vi "UHR-Fleezers Control (host) - 12.7c.vi"() -> ()   [LabVIEW 2012] (continued)
                n1635 = local write "Set Confocal Spot (X-Y)"(w2359) -> ()
                n1636 = local write "Set X Only"(w2359) -> ()
                n1637 = local write "Set Y Only"(w2359) -> ()
              }
            }
          }
          frame 3 {
            n1638 = local read "BD 2 Frequency 1 (MHz)"() -> (w2395:dbl)
            n1639 = local read "BD 1 Frequency 1 (MHz)"() -> (w2396:dbl)
            n1640 = local write "Manipulating Trap"(TRUE ("Manipulating Trap")) -> ()
            n1641 = local write "Coords"(T7 {"Horizontal"=0, "Vertical"=0} ("Coords")) -> ()
            n1642 = while {
              tunnel: w2401 -> [w2406]
              tunnel: w2399 -> [w2405]
              tunnel: w2397 -> [w2404]
              tunnel: w2396 -> [w2403]
              tunnel: w2395 -> [w2402]
              stop <- w2407 stop-if-true
              n1643 = event shown="[0] \"Pane\": Mouse Move" {
                selector: _ -> [_ _]
                dyn-events: _ -> [_ _]
                timeout: _ -> [_ _]
                tunnel: ["Force Manip Abort" w2471] -> w2407
                tunnel: w2406 -> [w2414 _]
                tunnel: w2405 -> [w2412 _]
                tunnel: w2404 -> [w2411 _]
                tunnel: w2403 -> [w2410 _]
                tunnel: w2402 -> [w2409 _]
                event Mouse Move {
                  n1644 = event-data() -> ("Time"=w2415:u32, "Coords"=w2416:T7)  [unwired: 3 out]
                  n1645 = Less?(x=w2415, y=w2414) -> (x < y?=w2413:bool)
                  n1646 = case "Makes sure old motion events prior to mouse click aren't used" shown="False" w2413 {
                    tunnel: w2416 -> [w2458 _]
                    tunnel: w2412 -> [w2459 _]
                    tunnel: w2411 -> [w2436 _]
                    tunnel: w2410 -> [w2432 _]
                    tunnel: w2409 -> [w2431 _]
                    frame False {
                      n1647 = Subtract(x=w2458, y=w2459) -> (x-y=w2457:T7)
                      "Coords" <- w2457
                      n1648 = local read "Y RF Frequency Limits (MHz)"() -> (w2417:T16)
                      n1649 = To Double Precision Float(number=w2457) -> (double precision float=w2456:cluster{"Horizontal":dbl, "Vertical":dbl})
                      n1650 = Multiply(x=cluster{"Horizontal":dbl, "Vertical":dbl} {"Horizontal"=-1.0, "Vertical"=1.0}, y="Manipulation Scaling") -> (x*y=w2452:cluster{"Horizontal":dbl, "Vertical":dbl})
                      n1651 = local read "X RF Frequency Limits (MHz)"() -> (w2418:T16)
                      n1652 = Multiply(x=w2456, y=w2452) -> (x*y=w2454:cluster{"Horizontal":dbl, "Vertical":dbl})
                      n1653 = Unbundle By Name(w2454) -> ("Horizontal"=w2449:dbl, "Vertical"=w2453:dbl)
                      n1654 = Unbundle By Name(w2417) -> ("Maximum"=w2420:dbl, "Minimum"=w2419:dbl)
                      n1655 = Boolean To (0,1)(Boolean="Manip. X?") -> (0, 1=w2447:i16)
                      n1656 = Boolean To (0,1)(Boolean="Manip. Y?") -> (0, 1=w2444:i16)
                      n1657 = local read "BD 1 Frequency 2 (MHz)"() -> (w2434:dbl)
                      n1658 = Multiply(x=w2453, y=w2444) -> (x*y=w2446:dbl)
                      n1659 = Multiply(x=w2447, y=w2449) -> (x*y=w2450:dbl)
                      n1660 = local read "BD 2 Frequency 2 (MHz)"() -> (w2433:dbl)
                      n1661 = Unbundle By Name(w2418) -> ("Maximum"=w2422:dbl, "Minimum"=w2421:dbl)
                      n1662 = Add(x=w2431, y=w2446) -> (x+y=w2424:dbl)
                      n1663 = Add(x=w2432, y=w2450) -> (x+y=w2426:dbl)
                      n1664 = In Range and Coerce(upper limit=w2422, x=w2426, lower limit=w2421) -> (coerced(x)=w2425:dbl)  [unwired: 1 out]
                      n1665 = In Range and Coerce(upper limit=w2420, x=w2424, lower limit=w2419) -> (coerced(x)=w2423:dbl)  [unwired: 1 out]
                      n1666 = Subtract(x=w2425, y=w2434) -> (x-y=w2443:dbl)
                      n1667 = Subtract(x=w2423, y=w2433) -> (x-y=w2442:dbl)
                      n1668 = Square(x=w2443) -> (x^2=w2441:dbl)
                      n1669 = Square(x=w2442) -> (x^2=w2440:dbl)
                      n1670 = Add(x=w2441, y=w2440) -> (x+y=w2439:dbl)
                      n1671 = Square Root(x=w2439) -> (sqrt(x)=w2435:dbl)
                      n1672 = In Range and Coerce(upper limit="Limit Max (MHz)", x=w2435, lower limit="Limit Min (MHz)") -> (In Range?=w2428:bool)  [unwired: 1 out]
                      n1673 = Not(x="Limits Enable") -> (.not. x?=w2427:bool)
                      n1674 = Or(x=w2428, y=w2427) -> (x .or. y?=w2429:bool)
                      n1675 = case shown="True" w2429 {
                        tunnel: w2436 -> [_ w2469]
                        tunnel: w2435 -> [_ w2460]
                        tunnel: w2425 -> [_ w2467]
                        tunnel: w2434 -> [_ w2466]
                        tunnel: w2423 -> [_ w2465]
                        tunnel: w2433 -> [_ w2464]
                        tunnel: w2418 -> [_ w2462]
                        tunnel: w2417 -> [_ w2461]
                        frame False {
                        }
                        frame True {
                          n1676 = local read "BD 1 Frequency 3 (MHz)"() -> (w2468:dbl)
                          n1677 = local read "BD 2 Frequency 3 (MHz)"() -> (w2463:dbl)
                          n1678 = local write "Trap Delta (MHz)"(w2460) -> ()
                          n1679 = call "set RF board frequency - interlace.vi"("Board 2 Frequency Limits"=w2461, "Board 1 Frequency Limits"=w2462, "FPGA VI Reference In"=w2469, "Board 2 Frequency 3 (MHz)"=w2463, "Board 1 Frequency 3 (MHz)"=w2468, "Board 2 Frequency 2 (MHz)"=w2464, "Board 2 Frequency 1 (MHz)"=w2465, "Board 1 Frequency 2 (MHz)"=w2466, "Board 1 Frequency 1  (MHz)"=w2467) -> ()  [unwired: 1 in, 2 out]
                          n1680 = local write "BD 2 Frequency 1 (MHz)"(w2465) -> ()
                          n1681 = local write "BD 1 Frequency 1 (MHz)"(w2467) -> ()
                        }
                      }
                    }
                    frame True {
                    }
                  }
                }
                event Mouse Up {
                  n1682 = event-data() -> ("Button"=w2470:u16)  [unwired: 8 out]
                  n1683 = case shown="3" w2470 {
                    tunnel: [FALSE TRUE] -> w2471
                    frame 0, Default {
                    }
                    frame 3 {
                      n1684 = local read "Trap Delta (MHz)"() -> (w2473:dbl)
                      n1685 = property on="Initial delta (MHz)" class="DigNum (strict)"("Val(Sgnl)"=w2473) -> ()  [unwired: 2 in, 2 out]
                      n1686 = local write "Manipulating Trap"(FALSE ("Manipulating Trap")) -> ()
                    }
                  }
                }
              }
            }
          }
        }
      }
      event Mouse Move {
        n1687 = event-data() -> ()  [unwired: 6 out]
      }
    }
    n1688 = local read "Stop All"() -> (w2289:bool)
    n1689 = node-c288() -> ()  [unwired: 2 out]
  }
  n1690 = timed-loop "Run Scripts, including: stage motion" {
    tunnel: w125 -> [w2484]
    tunnel: w124 -> [w2485]
    tunnel: [w2485] -> w123
    tunnel: [w2484] -> w122
    timing: w120 -> [_]
    timing-out: [_] -> w119
    tunnel: w106 -> [w2483]
    tunnel: w107 -> [w2482]
    tunnel: w78 -> [w2479]
    tunnel: w77 -> [w2478]
    tunnel: w76 -> [w2480]
    tunnel: w75 -> [w2481]
    tunnel: w13 -> [w2477]
    tunnel: w1 -> [w2476]
    stop <- w2486 stop-if-true
    n1691 = node-c288() -> ()  [unwired: 1 in, 1 out]
    n1692 = event shown="[22] \"Move in a Circle\": Value Change" {
      selector: _ -> [_ _ _ _ _ _ _ _ _ _ _ _ _ _ _ _ _ _ _ _ _ _ _ _]
      dyn-events: _ -> [_ _ _ _ _ _ _ _ _ _ _ _ _ _ _ _ _ _ _ _ _ _ _ _]
      timeout: _ -> [_ _ _ _ _ _ _ _ _ _ _ _ _ _ _ _ _ _ _ _ _ _ _ _]
      tunnel: ["Set Position" "Move to Position" _ _ _ _ _ _ "Read Harvard" _ _ _ _ _ _ "Got ADig bead" "Force FB Data\nScript" _ "Got DNA bead" "Take Stepping Data" _ "Take Detection Laser\nImage" _ _] -> _
      tunnel: [_ _ _ _ _ _ _ _ _ _ _ _ _ _ _ _ _ _ _ _ _ _ _ w3274] -> w2486
      tunnel: w2484 -> [w2504 w2512 w2525 w2555 _ _ _ _ _ w2671 w2711 w2792 w2821 w2953 w2979 _ w3015 _ _ _ _ _ _ _]
      tunnel: w2485 -> [w2505 w2513 w2526 w2556 _ _ _ _ _ w2672 w2712 w2793 w2822 w2954 w2980 _ w3016 _ _ _ _ _ _ _]
      tunnel: w2483 -> [_ _ _ _ _ _ _ _ w2656 _ _ _ _ _ _ _ _ _ _ _ _ _ _ _]
      tunnel: w2482 -> [_ _ _ _ _ _ _ _ w2655 _ _ _ _ _ _ _ _ _ _ _ _ _ _ _]
      tunnel: w2481 -> [_ _ _ _ _ _ _ _ _ _ _ _ _ _ _ _ _ _ _ _ _ _ _ _]
      tunnel: w2480 -> [_ _ _ _ _ _ _ _ _ _ _ _ _ _ _ _ _ _ _ _ _ _ _ _]
      tunnel: w2479 -> [_ _ _ _ _ _ _ _ _ _ _ _ _ _ _ _ _ _ _ _ _ _ _ _]
      tunnel: w2478 -> [_ _ _ _ _ _ _ _ _ _ _ _ _ _ _ _ _ _ _ _ _ _ _ _]
      tunnel: w2477 -> [_ _ _ _ w2583 w2611 w2635 w2646 _ _ _ _ _ _ _ _ _ _ _ _ _ _ _ w3273]
      tunnel: w2476 -> [_ _ _ _ _ _ _ _ _ _ _ _ _ _ _ _ _ _ _ _ _ _ w3174 _]
      event "Set Position", "Set Position 2", "Set Position 3", "Set Position 4", "Set Position 5", "Set Position 1": Value Change {
        n1693 = event-data() -> ()  [unwired: 1 in, 5 out]
        n1694 = Build Array("Set Position 1", "Set Position 2", "Set Position 3", "Set Position 4", "Set Position 5") -> (w2503:bool[])
        n1695 = Boolean Array To Number(Boolean array=w2503) -> (number=w2502:u32)
        n1696 = Logarithm Base 2(1:w2502) -> (0:w2494:dbl)
        n1697 = call "Read Stage Position.vi"("error in"=w2504, "VISA resource name in"=w2505) -> ("Current Position"=w2509:cluster{dbl, dbl, dbl}, "error out"=w2508:errorcluster)  [unwired: 2 out]
        n1698 = Decrement(x="Position") -> (x-1=w2492:dbl)
        n1699 = Greater Or Equal?(x=w2494, y=0.0) -> (x >= y?=w2495:bool)
        n1700 = Cluster To Array(cluster=w2509) -> (array=w2506:dbl[])
        n1701 = local write "Stage Control Serial Error"(w2508) -> ()
        n1702 = Select(t=w2494, s=w2495, f=w2492) -> (s? t:f=w2491:dbl)
        n1703 = Increment(x=w2491) -> (x+1=w2490:dbl)
        n1704 = Build Array (concatenate)(w2490, w2506) -> (w2489:dbl[])
        n1705 = Replace Array Subset(array="Saved Stage Positions", new element=w2489, index (row)=w2491) -> (w2507:dbl[][])  [unwired: 1 in]
        n1706 = local write "Saved Stage Positions"(w2507) -> ()
      }
      event "Move to Position": Value Change {
        n1707 = event-data() -> ()  [unwired: 1 in, 5 out]
        n1708 = flat-sequence {
          tunnel: w2513 -> [w2517]
          tunnel: w2512 -> [w2516]
          frame #0 {
            n1709 = local read "Saved Stage Positions"() -> (w2519:dbl[][])
            n1710 = local read "Position"() -> (w2518:dbl)
            n1711 = local write "Stage Moving"(TRUE ("Stage Moving")) -> ()
            n1712 = call "move to saved stage position.vi"("error in"=w2516, "Stage VISA resource name in"=w2517, "Position"=w2518, "Saved Stage Positions"=w2519) -> ("error out"=w2515:errorcluster)  [unwired: 1 out]
            n1713 = local write "Stage Control Serial Error"(w2515) -> ()
          }
          frame #1 {
            n1714 = call <vilib>:"Beep.vi"() -> ()  [unwired: 3 in, 9 out]
            n1715 = local write "Stage Moving"(FALSE ("Stage Moving")) -> ()
          }
        }
      }
      event "Move Cap. 1 (DNA Bottom)": Value Change {
        n1716 = event-data() -> ()  [unwired: 1 in, 5 out]
        n1717 = local write "Move Cap. 1 (DNA Bottom)"(FALSE ("Move Cap. 1 (DNA Right)")) -> ()
        n1718 = flat-sequence {
          tunnel: w2525 -> [w2528]
          tunnel: w2526 -> [w2529]
          tunnel: [w2529] -> w2523
          tunnel: [w2528] -> w2522
          tunnel: w2523 -> [w2531]
          tunnel: w2522 -> [w2530]
          frame #0 {
            n1719 = property on="Sample Channel\nFlow" class="Bool (strict)"("Val(Sgnl)"="Cap 1 Samp Flow ON") -> ()  [unwired: 2 in, 2 out]
          }
          frame #1 {
            n1720 = local read "Saved Stage Positions"() -> (w2541:dbl[][])
            n1721 = local write "Stage Moving"(TRUE ("Stage Moving")) -> ()
            n1722 = Array Subset(array=w2541, index (row)=0 ("index"), length (row)=1 ("length"), index (col)=1 ("index"), length (col)=3 ("length")) -> (w2538:dbl[][])
            n1723 = Reshape Array(w2538, 3 ("dimension size")) -> (w2536:dbl[])
            n1724 = Array To Cluster(array=w2536) -> (cluster=w2535:cluster{"[0]":dbl, "[1]":dbl, "[2]":dbl})
            n1725 = call "Set Stage Position.vi"("Position"=w2535, "error in"=w2530, "VISA resource name in"=w2531) -> ("error out"=w2534:errorcluster)  [unwired: 2 out]
            n1726 = local write "Stage Control Serial Error"(w2534) -> ()
          }
          frame #2 {
            n1727 = local write "Stage Moving"(FALSE ("Stage Moving")) -> ()
            n1728 = case shown="True" "Cap 1 Flow ON" {
              frame False {
              }
              frame True {
                n1729 = property on="Inject Pump 1" class="Bool (strict)"("Val(Sgnl)"=TRUE ("Value (Signaling)")) -> ()  [unwired: 2 in, 2 out]
              }
            }
            n1730 = call <vilib>:"Beep.vi"() -> ()  [unwired: 3 in, 9 out]
          }
          frame #3 {
            n1731 = property on="Sample Channel\nFlow" class="Bool (strict)"("Val(Sgnl)"=FALSE ("Value (Signaling)")) -> ()  [unwired: 2 in, 2 out]
            n1732 = local read "Cap. 2 BD T1?\n(ADig T1, DNA T2)"() -> (w2548:bool)
            n1733 = case shown="True" w2548 {
              tunnel: "Cap 1 T ON" -> [w2550 w2551]
              frame False {
                n1734 = property on="Trap 1 (ON/OFF)" class="Bool (strict)"("Val(Sgnl)"=w2550) -> ()  [unwired: 2 in, 2 out]
              }
              frame True {
                n1735 = property on="Trap 2 (ON/OFF)" class="Bool (strict)"("Val(Sgnl)"=w2551) -> ()  [unwired: 2 in, 2 out]
              }
            }
            n1736 = property on="Got DNA bead" class="Bool"("Key Focus"=TRUE) -> ()  [unwired: 2 in, 2 out]
          }
        }
      }
      event "Move Cap. 2 (ADig Top)": Value Change {
        n1737 = event-data() -> ()  [unwired: 1 in, 5 out]
        n1738 = local write "Move Cap. 2 (ADig Top)"(FALSE ("Move Cap. 2 (ADig Left)")) -> ()
        n1739 = flat-sequence {
          tunnel: w2555 -> [w2558]
          tunnel: w2556 -> [w2559]
          tunnel: [w2559] -> w2553
          tunnel: [w2558] -> w2552
          tunnel: w2553 -> [w2562]
          tunnel: w2552 -> [w2561]
          frame #0 {
            n1740 = property on="Sample Channel\nFlow" class="Bool (strict)"("Val(Sgnl)"="Cap 2 Samp Flow ON") -> ()  [unwired: 2 in, 2 out]
          }
          frame #1 {
            w2560 = FALSE ("Value (Signaling)")
            n1741 = local read "Saved Stage Positions"() -> (w2572:dbl[][])
            n1742 = local write "Stage Moving"(TRUE ("Stage Moving")) -> ()
            n1743 = Array Subset(array=w2572, index (row)=1 ("index"), length (row)=1 ("length"), index (col)=1 ("index"), length (col)=3 ("length")) -> (w2569:dbl[][])
            n1744 = Reshape Array(w2569, 3 ("dimension size")) -> (w2567:dbl[])
            n1745 = property on="Trap 1 (ON/OFF)" class="Bool (strict)"("Val(Sgnl)"=w2560) -> ()  [unwired: 2 in, 2 out]
            n1746 = property on="Trap 1 (ON/OFF)" class="Bool (strict)"("Val(Sgnl)"=w2560) -> ()  [unwired: 2 in, 2 out]
            n1747 = Array To Cluster(array=w2567) -> (cluster=w2566:cluster{"[0]":dbl, "[1]":dbl, "[2]":dbl})
            n1748 = call "Set Stage Position.vi"("Position"=w2566, "error in"=w2561, "VISA resource name in"=w2562) -> ("error out"=w2565:errorcluster)  [unwired: 2 out]
            n1749 = local write "Stage Control Serial Error"(w2565) -> ()
          }
          frame #2 {
            n1750 = local write "Stage Moving"(FALSE ("Stage Moving")) -> ()
            n1751 = call <vilib>:"Beep.vi"() -> ()  [unwired: 3 in, 9 out]
            n1752 = case shown="True" "Cap 2 Flow ON" {
              frame False {
              }
              frame True {
                n1753 = property on="Inject Pump 3" class="Bool (strict)"("Val(Sgnl)"=TRUE ("Value (Signaling)")) -> ()  [unwired: 2 in, 2 out]
              }
            }
          }
          frame #3 {
            n1754 = property on="Sample Channel\nFlow" class="Bool (strict)"("Val(Sgnl)"=FALSE ("Value (Signaling)")) -> ()  [unwired: 2 in, 2 out]
            n1755 = case shown="False" "Cap. 2 BD T1?\n(ADig T1, DNA T2)" {
              tunnel: "Cap 2 T ON" -> [w2581 w2582]
              frame False {
                n1756 = property on="Trap 2 (ON/OFF)" class="Bool (strict)"("Val(Sgnl)"=w2581) -> ()  [unwired: 2 in, 2 out]
              }
              frame True {
                n1757 = property on="Trap 1 (ON/OFF)" class="Bool (strict)"("Val(Sgnl)"=w2582) -> ()  [unwired: 2 in, 2 out]
              }
            }
            n1758 = property on="Got ADig bead" class="Bool"("Key Focus"=TRUE) -> ()  [unwired: 2 in, 2 out]
          }
        }
      }
      event "Initialize Blue Laser": Value Change {
        n1759 = event-data() -> ()  [unwired: 1 in, 5 out]
        n1760 = flat-sequence {
          tunnel: w2583 -> [w2602]
          frame #0 {
            n1761 = Concatenate Strings("slmp ", "Blue Laser\nModulation\nPower (mW)") -> (w2601:string)
            n1762 = call "serial write macro.vi"("String"=w2601, "Delay (ms)"="Delay (ms)", "VISA resource name"=w2602) -> ("read buffer"=w2590:string, "error out"=w2591:errorcluster, "VISA resource name out"=w2598:refnum<visa-resource-name>)
            n1763 = local write "read blue buffer"(w2590) -> ()
            n1764 = local write "Blue Error Out"(w2591) -> ()
            n1765 = call "serial write macro.vi"("String"="sdmes 1", "Delay (ms)"="Delay (ms)", "VISA resource name"=w2598) -> ("read buffer"=w2588:string, "error out"=w2589:errorcluster, "VISA resource name out"=w2596:refnum<visa-resource-name>)
            n1766 = local write "Blue Error Out"(w2589) -> ()
            n1767 = local write "read blue buffer"(w2588) -> ()
            n1768 = call "serial write macro.vi"("String"="sames 1", "Delay (ms)"="Delay (ms)", "VISA resource name"=w2596) -> ("read buffer"=w2585:string, "error out"=w2587:errorcluster, "VISA resource name out"=w2593:refnum<visa-resource-name>)
            n1769 = local write "read blue buffer"(w2585) -> ()
            n1770 = local write "Blue Error Out"(w2587) -> ()
            n1771 = call "serial write macro.vi"("String"="l1", "Delay (ms)"="Delay (ms)", "VISA resource name"=w2593) -> ("read buffer"=w2584:string, "error out"=w2586:errorcluster)  [unwired: 1 out]
            n1772 = local write "read blue buffer"(w2584) -> ()
            n1773 = local write "Blue Error Out"(w2586) -> ()
          }
          frame #1 {
            n1774 = local write "Initialize Blue Laser"(FALSE ("Initialize")) -> ()
          }
        }
      }
      event "Blue Laser Modluation Mode": Value Change {
        # "Changes the type of modulation for the blue laser"
        n1775 = event-data() -> ()  [unwired: 1 in, 5 out]
        n1776 = case shown="\"Constant Power\"" "Blue Laser Modluation Mode" {
          tunnel: ["sdmes 1" w2620 "sdmes 1" "sdmes 0"] -> w2605
          tunnel: ["sames 1" "cp" "sames 0" "sames 1"] -> w2604
          frame "Digital + Analog", Default {
          }
          frame "Constant Power" {
            n1777 = local read "Blue Laser\nModulation\nPower (mW)"() -> (w2623:string)
            n1778 = Decimal String To Number(string=w2623) -> (number=w2619:i32)  [unwired: 2 in, 1 out]
            n1779 = Divide(x=w2619, y=1000) -> (x/y=w2617:dbl)
            n1780 = Number To Fractional String(number=w2617) -> (F-format string=w2618:string)  [unwired: 3 in]
            n1781 = Concatenate Strings("p ", w2618) -> (w2620:string)
          }
          frame "Digital Only" {
          }
          frame "Analog Only" {
          }
        }
        n1782 = local read "Delay (ms)"() -> (w2614:i32)
        n1783 = call "serial write macro.vi"("String"=w2605, "Delay (ms)"=w2614, "VISA resource name"=w2611) -> ("read buffer"=w2612:string, "error out"=w2613:errorcluster, "VISA resource name out"=w2606:refnum<visa-resource-name>)
        n1784 = local write "read blue buffer"(w2612) -> ()
        n1785 = local write "Blue Error Out"(w2613) -> ()
        n1786 = local read "Delay (ms)"() -> (w2609:i32)
        n1787 = call "serial write macro.vi"("String"=w2604, "Delay (ms)"=w2609, "VISA resource name"=w2606) -> ("read buffer"=w2607:string, "error out"=w2608:errorcluster)  [unwired: 1 out]
        n1788 = local write "Blue Error Out"(w2608) -> ()
        n1789 = local write "read blue buffer"(w2607) -> ()
      }
      event "Blue Laser\nModulation\nPower (mW)": Value Change {
        n1790 = event-data() -> ()  [unwired: 1 in, 5 out]
        n1791 = local read "Blue Laser\nModulation\nPower (mW)"() -> (w2630:string)
        n1792 = local read "Blue Laser Modluation Mode"() -> (w2631:string)
        n1793 = case shown="\"Constant Power\"" w2631 {
          tunnel: w2630 -> [w2637 w2644]
          tunnel: [w2636 w2643] -> w2629
          frame "Constant Power" {
            # "Different command to change constant power instead of modulation power"
            n1794 = Decimal String To Number(string=w2637) -> (offset past number=w2642:i32)  [unwired: 2 in, 1 out]
            n1795 = Divide(x=w2642, y=1000) -> (x/y=w2640:dbl)
            n1796 = Number To Fractional String(number=w2640) -> (F-format string=w2638:string)  [unwired: 3 in]
            n1797 = Concatenate Strings("p ", w2638) -> (w2636:string)
          }
          frame Default {
            n1798 = Concatenate Strings("slmp ", w2644) -> (w2643:string)
          }
        }
        n1799 = local read "Delay (ms)"() -> (w2634:i32)
        n1800 = call "serial write macro.vi"("String"=w2629, "Delay (ms)"=w2634, "VISA resource name"=w2635) -> ("read buffer"=w2633:string, "error out"=w2632:errorcluster)  [unwired: 1 out]
        n1801 = local write "Blue Error Out"(w2632) -> ()
        n1802 = local write "read blue buffer"(w2633) -> ()
      }
      event "Send string\nto Blue Laser": Value Change {
        n1803 = event-data() -> ()  [unwired: 1 in, 5 out]
        n1804 = flat-sequence {
          tunnel: w2646 -> [w2651]
          frame #0 {
            n1805 = local read "Delay (ms)"() -> (w2648:i32)
            n1806 = call "serial write macro.vi"("String"="command string", "Delay (ms)"=w2648, "VISA resource name"=w2651) -> ("read buffer"=w2649:string, "error out"=→"Blue Error Out":errorcluster)  [unwired: 1 out]
            "read blue buffer" <- w2649
            n1807 = String Length(string=w2649) -> (length=→"length":i32)
            "command string sent" <- "command string"
          }
          frame #1 {
            n1808 = local write "Send string\nto Blue Laser"(FALSE ("Send string")) -> ()
          }
        }
      }
      event "Read Harvard": Value Change {
        n1809 = event-data() -> ()  [unwired: 1 in, 5 out]
        n1810 = Concatenate Strings("write buffer", "\r") -> (w2658:string)
        n1811 = VISA Write(VISA resource name=w2656, write buffer=w2658, error in (no error)=w2655) -> (VISA resource name out=w2667:refnum<visa-resource-name>, error out=w2666:errorcluster)  [unwired: 1 out]
        n1812 = stacked-sequence {
          tunnel: [w2670] -> w2665
          tunnel: w2667 -> [w2670]
          tunnel: w2666 -> [w2669]
          tunnel: [w2669] -> w2660
          frame #0 {
            n1813 = Wait (ms)(milliseconds to wait=50) -> ()  [unwired: 1 out]
          }
        }
        n1814 = property class="Instr"(reference=w2665, error in=w2660) -> (reference out=w2664:refnum<visa-resource-name>, error out=w2662:errorcluster, "Serial Settings:Number of Bytes at Serial Port"=w2663:u32)
        "Serial Settings:Number of Bytes at Serial Port" <- w2663
        n1815 = VISA Read(VISA resource name=w2664, byte count=w2663, error in (no error)=w2662) -> (read buffer=w2661:string)  [unwired: 3 out]
        "read buffer" <- w2661
        n1816 = Fract/Exp String To Number(string=w2661) -> ()  [unwired: 5 out]
      }
      event "+z", "-z": Value Change {
        n1817 = event-data() -> ()  [unwired: 1 in, 5 out]
        n1818 = flat-sequence {
          tunnel: w2671 -> [w2693]
          tunnel: w2672 -> [w2673]
          frame #0 {
            n1819 = call "Read Stage Position.vi"("error in"=w2693, "VISA resource name in"=w2673) -> ("Current Position"=w2678:cluster{dbl, dbl, dbl}, "error out"=w2691:errorcluster, "VISA resource name out"=w2692:refnum<visa-resource-name>)  [unwired: 1 out]
            n1820 = local read "Saved Stage Positions"() -> (w2702:dbl[][])
            n1821 = Divide(x="z nudge increment (um)", y=1000.0) -> (x/y=w2690:dbl)
            n1822 = Boolean To (0,1)(Boolean="+z") -> (0, 1=w2682:i16)
            n1823 = Boolean To (0,1)(Boolean="-z") -> (0, 1=w2683:i16)
            n1824 = Array Subset(array=w2702, index (row)=1 ("index"), length (row)=1 ("length"), index (col)=1 ("index"), length (col)=3 ("length")) -> (w2699:dbl[][])
            n1825 = Multiply(x=w2682, y=w2690) -> (x*y=w2686:dbl)
            n1826 = Multiply(x=w2683, y=w2690) -> (x*y=w2684:dbl)
            n1827 = Unbundle(w2678) -> (w2676:dbl, w2675:dbl, w2679:dbl)
            n1828 = Negate(x=w2684) -> (-x=w2685:dbl)
            n1829 = Reshape Array(w2699, 3 ("dimension size")) -> (w2697:dbl[])
            n1830 = Add(x=w2686, y=w2685) -> (x+y=w2687:dbl)
            n1831 = Array To Cluster(array=w2697) -> ()  [unwired: 1 out]
            n1832 = Add(x=w2687, y=w2679) -> (x+y=w2677:dbl)
            n1833 = Bundle(cluster=w2678, w2676, w2675, w2677) -> (w2674:cluster{dbl, dbl, dbl})
            n1834 = call "Set Stage Position.vi"("Position"=w2674, "error in"=w2691, "VISA resource name in"=w2692) -> ("error out"=w2696:errorcluster)  [unwired: 2 out]
            n1835 = local write "Stage Moving"(TRUE ("Stage Moving")) -> ()
            n1836 = local write "Stage Control Serial Error"(w2696) -> ()
          }
          frame #1 {
            n1837 = local write "Stage Moving"(FALSE ("Stage Moving")) -> ()
            n1838 = call <vilib>:"Beep.vi"() -> ()  [unwired: 3 in, 9 out]
          }
        }
      }
      event "Cal/Data Acq. Spot": Value Change {
        n1839 = event-data() -> ()  [unwired: 1 in, 5 out]
        n1840 = flat-sequence {
          tunnel: w2711 -> [w2715]
          tunnel: w2712 -> [w2716]
          tunnel: [w2716] -> w2708
          tunnel: [w2715] -> w2707
          tunnel: w2708 -> [w2721]
          tunnel: w2707 -> [w2720]
          tunnel: ["Cal @ (MHz)"] -> w2705
          tunnel: [w2725] -> w2709
          tunnel: w2705 -> [w2725]
          tunnel: w2709 -> [w2734]
          tunnel: ["W/ Offset 1"] -> w2706
          tunnel: w2709 -> [w2755]
          tunnel: w2706 -> [w2753]
          frame #0 {
            n1841 = property on="Sample Channel\nFlow" class="Bool (strict)"("Val(Sgnl)"="Daq spot flow on") -> ()  [unwired: 2 in, 2 out]
            n1842 = Wait (ms)(milliseconds to wait=u32 250) -> ()  [unwired: 1 out]
          }
          frame #1 {
            n1843 = local read "Saved Stage Positions"() -> (w2718:dbl[][])
            n1844 = property on="Trap Delta (MHz)" class="DigNum (strict)"("Val(Sgnl)"="Cal @ (MHz)") -> ()  [unwired: 2 in, 2 out]
            n1845 = local write "Stage Moving"(TRUE ("Stage Moving")) -> ()
            n1846 = call "move to saved stage position.vi"("error in"=w2720, "Stage VISA resource name in"=w2721, "Position"="Cal Stage Position", "Saved Stage Positions"=w2718) -> ("error out"=w2719:errorcluster)  [unwired: 1 out]
            n1847 = local write "Stage Control Serial Error"(w2719) -> ()
          }
          frame #2 {
            n1848 = local write "Stage Moving"(FALSE ("Stage Moving")) -> ()
            n1849 = property on="Sample Channel\nFlow" class="Bool (strict)"("Val(Sgnl)"="Flow ON during cal?") -> ()  [unwired: 2 in, 2 out]
            n1850 = call <vilib>:"Beep.vi"() -> ()  [unwired: 3 in, 9 out]
          }
          frame #3 {
            n1851 = Wait (ms)(milliseconds to wait=u32 1000) -> ()  [unwired: 1 out]
          }
          frame #4 {
            n1852 = property on="Save Calibration" class="Bool (strict)"("Val(Sgnl)"=TRUE ("Value (Signaling)")) -> ()  [unwired: 2 in, 2 out]
          }
          frame #5 {
            n1853 = Wait (ms)(milliseconds to wait=u32 2000) -> ()  [unwired: 1 out]
          }
          frame #6 {
            # "Check to see if \nsaving done"
            n1854 = while {
              stop <- w2730 stop-if-true
              n1855 = local read "Saving..."() -> (w2731:bool)
              n1856 = Wait (ms)(milliseconds to wait=u32 100) -> ()  [unwired: 1 out]
              n1857 = Not(x=w2731) -> (.not. x?=w2730:bool)
            }
          }
          frame #7 {
            n1858 = case shown="True" "W/ Offset 1" {
              tunnel: w2734 -> [_ w2735]
              frame False {
              }
              frame True {
                n1859 = stacked-sequence {
                  tunnel: w2735 -> [_ _ _ _ _ _ _ w2752]
                  frame #0 {
                    n1860 = property on="Trap Delta (MHz)" class="DigNum (strict)"("Val(Sgnl)"="Offset 1 Start (MHz)") -> ()  [unwired: 2 in, 2 out]
                    n1861 = Replace Array Subset(array=u32[] [0] ("Index Values"), new element="Offset 1 Set", index=0) -> (w2736:u32[])
                    n1862 = property on="Saved AOD Raster Scan Parameter Sets" class="Arr (strict)"("Index Values"=w2736) -> ()  [unwired: 2 in, 2 out]
                  }
                  frame #1 {
                    n1863 = Wait (ms)(milliseconds to wait=u32 200) -> ()  [unwired: 1 out]
                  }
                  frame #2 {
                    n1864 = property on="Load parameters" class="Bool (strict)"("Val(Sgnl)"=TRUE ("Value (Signaling)")) -> ()  [unwired: 2 in, 2 out]
                  }
                  frame #3 {
                    n1865 = Wait (ms)(milliseconds to wait=u32 200) -> ()  [unwired: 1 out]
                  }
                  frame #4 {
                    n1866 = property on="Trap Raster Scan" class="Bool (strict)"("Val(Sgnl)"=TRUE ("Value (Signaling)")) -> ()  [unwired: 2 in, 2 out]
                  }
                  frame #5 {
                    n1867 = Wait (ms)(milliseconds to wait=u32 2000) -> ()  [unwired: 1 out]
                  }
                  frame #6 {
                    n1868 = while {
                      stop <- w2749 stop-if-true
                      n1869 = local read "Raster Scanning..."() -> (w2751:bool)
                      n1870 = local read "Saving..."() -> (w2747:bool)
                      n1871 = Wait (ms)(milliseconds to wait=u32 100) -> ()  [unwired: 1 out]
                      n1872 = Not(x=w2747) -> (.not. x?=w2746:bool)
                      n1873 = Not(x=w2751) -> (.not. x?=w2748:bool)
                      n1874 = And(x=w2748, y=w2746) -> (x .and. y?=w2749:bool)
                    }
                  }
                  frame #7 {
                    n1875 = property on="Trap Delta (MHz)" class="DigNum (strict)"("Val(Sgnl)"=w2752) -> ()  [unwired: 2 in, 2 out]
                  }
                }
              }
            }
          }
          frame #8 {
            n1876 = local read "Save ave N"() -> (w2754:dbl)
            n1877 = case shown="False" "W/ Offset 2" {
              tunnel: w2755 -> [_ w2762]
              tunnel: w2754 -> [_ w2761]
              tunnel: w2753 -> [w2757 _]
              frame False {
                n1878 = case shown="False" w2757 {
                  frame False {
                    n1879 = Multiply(x="Cal read wait (s)", y=u32 1000 ("milliseconds to wait")) -> (x*y=w2759:u32)
                    n1880 = Wait (ms)(milliseconds to wait=w2759) -> ()  [unwired: 1 out]
                  }
                  frame True {
                  }
                }
              }
              frame True {
                n1881 = stacked-sequence {
                  tunnel: w2762 -> [_ _ _ _ _ _ _ _ _ w2783 _ _]
                  tunnel: w2761 -> [_ _ _ _ _ _ _ _ _ w2781 _ _]
                  frame #0 {
                    n1882 = property on="Save ave N" class="DigNum (strict)"("Val(Sgnl)"=1.0 ("Value (Signaling)")) -> ()  [unwired: 2 in, 2 out]
                  }
                  frame #1 {
                    n1883 = Wait (ms)(milliseconds to wait=u32 500) -> ()  [unwired: 1 out]
                  }
                  frame #2 {
                    n1884 = property on="Trap Delta (MHz)" class="DigNum (strict)"("Val(Sgnl)"="Offset 2 Start (MHz)") -> ()  [unwired: 2 in, 2 out]
                    n1885 = Replace Array Subset(array=u32[] [0] ("Index Values"), new element="Offset 2 Set", index=0) -> (w2767:u32[])
                    n1886 = property on="Saved AOD Raster Scan Parameter Sets" class="Arr (strict)"("Index Values"=w2767) -> ()  [unwired: 2 in, 2 out]
                  }
                  frame #3 {
                    n1887 = Wait (ms)(milliseconds to wait=u32 500) -> ()  [unwired: 1 out]
                  }
                  frame #4 {
                    n1888 = property on="Load parameters" class="Bool (strict)"("Val(Sgnl)"=TRUE ("Value (Signaling)")) -> ()  [unwired: 2 in, 2 out]
                  }
                  frame #5 {
                    n1889 = Wait (ms)(milliseconds to wait=u32 500) -> ()  [unwired: 1 out]
                  }
                  frame #6 {
                    n1890 = property on="Trap Raster Scan" class="Bool (strict)"("Val(Sgnl)"=TRUE ("Value (Signaling)")) -> ()  [unwired: 2 in, 2 out]
                  }
                  frame #7 {
                    n1891 = Wait (ms)(milliseconds to wait=u32 2000) -> ()  [unwired: 1 out]
                  }
                  frame #8 {
                    n1892 = while {
                      stop <- w2776 stop-if-true
                      n1893 = local read "Raster Scanning..."() -> (w2779:bool)
                      n1894 = local read "Saving..."() -> (w2777:bool)
                      n1895 = Wait (ms)(milliseconds to wait=u32 100) -> ()  [unwired: 1 out]
                      n1896 = Not(x=w2777) -> (.not. x?=w2775:bool)
                      n1897 = Not(x=w2779) -> (.not. x?=w2778:bool)
                      n1898 = And(x=w2778, y=w2775) -> (x .and. y?=w2776:bool)
                    }
                  }
                  frame #9 {
                    n1899 = property on="Trap Delta (MHz)" class="DigNum (strict)"("Val(Sgnl)"=w2783) -> ()  [unwired: 2 in, 2 out]
                    n1900 = property on="Saved AOD Raster Scan Parameter Sets" class="Arr (strict)"("Index Values"=u32[] [0]) -> ()  [unwired: 2 in, 2 out]
                    n1901 = property on="Save ave N" class="DigNum (strict)"("Val(Sgnl)"=w2781) -> ()  [unwired: 2 in, 2 out]
                  }
                  frame #10 {
                    n1902 = Wait (ms)(milliseconds to wait=u32 500) -> ()  [unwired: 1 out]
                  }
                  frame #11 {
                    n1903 = property on="Load parameters" class="Bool (strict)"("Val(Sgnl)"=TRUE ("Value (Signaling)")) -> ()  [unwired: 2 in, 2 out]
                  }
                }
              }
            }
          }
          frame #9 {
            n1904 = property on="Read Cal" class="Bool (strict)"("Val(Sgnl)"=TRUE ("Value (Signaling)")) -> ()  [unwired: 2 in, 2 out]
          }
          frame #10 {
            n1905 = Wait (ms)(milliseconds to wait=u32 1000) -> ()  [unwired: 1 out]
          }
          frame #11 {
            n1906 = property on="Fish for Tether" class="Bool (strict)"("Val(Sgnl)"=TRUE ("Value (Signaling)")) -> ()  [unwired: 2 in, 2 out]
          }
        }
        n1907 = local write "Cal/Data Acq. Spot"(FALSE ("Cal/Data Acq. Spot")) -> ()
      }
      event "Dump Beads": Value Change {
        n1908 = event-data() -> ()  [unwired: 1 in, 5 out]
        n1909 = flat-sequence {
          tunnel: ["Dump spot flow on?"] -> w2789
          tunnel: [w2800] -> w2790
          tunnel: w2789 -> [w2800]
          tunnel: w2793 -> [w2805]
          tunnel: w2792 -> [w2804]
          tunnel: [w2802] -> w2791
          tunnel: w2790 -> [w2802]
          tunnel: w2791 -> [w2815]
          frame #0 {
            w2794 = FALSE ("Value (Signaling)")
            n1910 = local read "Saving..."() -> (w2796:bool)
            n1911 = local write "Dump Beads"(FALSE ("Dump Beads")) -> ()
            n1912 = property on="Inject Pump 3" class="Bool (strict)"("Val(Sgnl)"=w2794) -> ()  [unwired: 2 in, 2 out]
            n1913 = property on="Inject Pump 1" class="Bool (strict)"("Val(Sgnl)"=w2794) -> ()  [unwired: 2 in, 2 out]
            n1914 = local write "Stop Saving"(w2796) -> ()
          }
          frame #1 {
            w2797 = FALSE ("Fl. Triggered...")
            n1915 = case shown="True" "Dump spot flow on?" {
              frame False {
              }
              frame True {
                n1916 = property on="Sample Channel\nFlow" class="Bool (strict)"("Val(Sgnl)"=TRUE ("Stage Moving")) -> ()  [unwired: 2 in, 2 out]
              }
            }
            n1917 = local write "Fl. Triggered..."(w2797) -> ()
            n1918 = local write "Tether"(w2797) -> ()
            n1919 = property on="Green Laser ON" class="Bool (strict)"("Val(Sgnl)"=w2797) -> ()  [unwired: 2 in, 2 out]
            n1920 = property on="Trap Pos. FB ON" class="Bool (strict)"("Val(Sgnl)"=w2797) -> ()  [unwired: 2 in, 2 out]
            n1921 = property on="Trap Trig. Fl." class="Bool (strict)"("Val(Sgnl)"=w2797) -> ()  [unwired: 2 in, 2 out]
            n1922 = property on="Fl. Triggered..." class="Bool (strict)"("Val(Sgnl)"=w2797) -> ()  [unwired: 2 in, 2 out]
            n1923 = property on="Dip for Protein" class="Bool (strict)"("Val(Sgnl)"=w2797) -> ()  [unwired: 2 in, 2 out]
            n1924 = property on="Pause dwell" class="Bool (strict)"("Val(Sgnl)"=w2797) -> ()  [unwired: 2 in, 2 out]
          }
          frame #2 {
            n1925 = property on="Trap Pos. FB Offset Factor" class="DigNum (strict)"("Val(Sgnl)"=i64 0 ("Value (Signaling)")) -> ()  [unwired: 2 in, 2 out]
          }
          frame #3 {
            n1926 = local read "Saved Stage Positions"() -> (w2806:dbl[][])
            n1927 = local write "Stage Moving"(TRUE ("Stage Moving")) -> ()
            n1928 = Array Subset(array=w2806, index (row)=3 ("index"), length (row)=1 ("length"), index (col)=1 ("index"), length (col)=3 ("length")) -> (w2811:dbl[][])
            n1929 = Reshape Array(w2811, 3 ("dimension size")) -> (w2809:dbl[])
            n1930 = Array To Cluster(array=w2809) -> (cluster=w2808:cluster{"[0]":dbl, "[1]":dbl, "[2]":dbl})
            n1931 = call "Set Stage Position.vi"("Position"=w2808, "error in"=w2804, "VISA resource name in"=w2805) -> ()  [unwired: 3 out]
          }
          frame #4 {
            w2816 = FALSE ("Value (Signaling)")
            n1932 = case shown="True" w2815 {
              frame False {
              }
              frame True {
                n1933 = property on="Sample Channel\nFlow" class="Bool (strict)"("Val(Sgnl)"=FALSE ("Stage Moving")) -> ()  [unwired: 2 in, 2 out]
              }
            }
            n1934 = property on="Trap 1 (ON/OFF)" class="Bool (strict)"("Val(Sgnl)"=w2816) -> ()  [unwired: 2 in, 2 out]
            n1935 = property on="Trap 2 (ON/OFF)" class="Bool (strict)"("Val(Sgnl)"=w2816) -> ()  [unwired: 2 in, 2 out]
            n1936 = call <vilib>:"Beep.vi"() -> ()  [unwired: 3 in, 9 out]
          }
          frame #5 {
            n1937 = property on="Move Cap. 2 (ADig Top)" class="Bool (strict)"("Val(Sgnl)"=TRUE ("Value (Signaling)")) -> ()  [unwired: 2 in, 2 out]
            n1938 = property on="Tab Control" class="TabCtl (strict)"("Val(Sgnl)"=T33."Status" ("Value (Signaling)")) -> ()  [unwired: 2 in, 2 out]
          }
        }
      }
      event "Dip for Protein": Value Change {
        n1939 = event-data() -> ()  [unwired: 1 in, 5 out]
        n1940 = case shown="True" "Dip for Protein" {
          tunnel: w2822 -> [_ w2824]
          tunnel: w2821 -> [_ w2823]
          frame False {
          }
          frame True {
            n1941 = while {
              tunnel: w2824 -> [w2835]
              tunnel: w2823 -> [w2834]
              i -> [w2829]
              stop <- w2831 stop-if-true
              n1942 = Increment(x=w2829) -> (x+1=→"Dip #":i32)
              n1943 = flat-sequence {
                tunnel: w2834 -> [w2846]
                tunnel: w2835 -> [w2847]
                tunnel: [w2847] -> w2839
                tunnel: [w2846] -> w2838
                tunnel: [w2840] -> w2825
                tunnel: [w2852] -> w2833
                tunnel: [w2853] -> w2832
                tunnel: w2839 -> [w2854]
                tunnel: w2838 -> [w2855]
                tunnel: [w2850] -> w2826
                tunnel: w2825 -> [w2850]
                tunnel: [w2863] -> w2837
                tunnel: w2833 -> [w2863]
                tunnel: [w2862] -> w2836
                tunnel: w2832 -> [w2862]
                tunnel: [w2859] -> w2830
                tunnel: [w2858] -> w2827
                tunnel: w2826 -> [w2858]
                tunnel: w2836 -> [w2883]
                tunnel: w2837 -> [w2884]
                tunnel: w2830 -> [w2885]
                tunnel: w2827 -> [w2882]
                tunnel: [w2941] -> w2831
                frame #0 {
                  n1944 = local read "Trap Pos. FB ON"() -> (w2840:bool)
                  n1945 = Compound Arithmetic op=AND("Flow ON\nduring dip?", "FB OFF when \nflow ON", w2840) -> (w2841:bool)
                  n1946 = case shown="True" "Move trap \nbefore dip move?" {
                    frame False {
                    }
                    frame True {
                      n1947 = property on="Trap Delta (MHz)" class="DigNum (strict)"("Val(Sgnl)"="Dipping Delta (MHz)") -> ()  [unwired: 2 in, 2 out]
                    }
                  }
                  n1948 = property on="Green Laser ON" class="Bool (strict)"("Val(Sgnl)"="Green ON\nbefore dip?") -> ()  [unwired: 2 in, 2 out]
                  n1949 = property on="Sample Channel\nFlow" class="Bool (strict)"("Val(Sgnl)"="Flow ON\nduring dip?") -> ()  [unwired: 2 in, 2 out]
                  n1950 = case shown="True" w2841 {
                    frame False {
                    }
                    frame True {
                      n1951 = property on="Trap Pos. FB ON" class="Bool (strict)"("Val(Sgnl)"=FALSE ("Value (Signaling)")) -> ()  [unwired: 2 in, 2 out]
                    }
                  }
                }
                frame #1 {
                  n1952 = local read "Saved Stage Positions"() -> (w2857:dbl[][])
                  n1953 = local write "Cancel dwell"(FALSE ("Cancel dwell")) -> ()
                  n1954 = call "move to saved stage position.vi"("error in"=w2855, "Stage VISA resource name in"=w2854, "Position"="Dip Stage \nPosition", "Saved Stage Positions"=w2857) -> ("VISA resource name out"=w2852:refnum<visa-resource-name>, "error out"=w2853:errorcluster)
                }
                frame #2 {
                  n1955 = node-c288() -> (w2861:T23)  [unwired: 4 in]
                  n1956 = timed-loop {
                    timing: w2861 -> [_]
                    timing-out: [_] -> w2860
                    tunnel: [w2867] -> w2859
                    i -> [w2864]
                    stop <- w2868 stop-if-true
                    n1957 = node-c288() -> ()  [unwired: 1 in, 1 out]
                    n1958 = Greater Or Equal?(x=w2864, y="Dip Duration (s)") -> (x >= y?=w2876:bool)
                    n1959 = local read "Dip for Protein"() -> (w2869:bool)
                    n1960 = local read "Dump Beads"() -> (w2866:bool)
                    n1961 = local read "Cancel dwell"() -> (w2875:bool)
                    n1962 = local read "Pause dwell"() -> (w2872:bool)
                    n1963 = Not(x=w2869) -> (.not. x?=w2874:bool)
                    n1964 = Compound Arithmetic op=OR(w2875, w2876, w2874) -> (w2873:bool)
                    n1965 = Select(t=FALSE, s=w2872, f=w2873) -> (s? t:f=w2870:bool)
                    n1966 = Not(x=w2866) -> (.not. x?=w2865:bool)
                    n1967 = node-c288() -> ()  [unwired: 1 in, 1 out]
                    n1968 = And(x=w2869, y=w2865) -> (x .and. y?=w2867:bool)
                    n1969 = Or(x=w2870, y=w2866) -> (x .or. y?=w2868:bool)
                    "Dip Time (s)" <- w2864
                  }
                  n1970 = node-c288(w2860) -> ()  [unwired: 1 out]
                }
                frame #3 {
                  n1971 = case shown="True" w2885 {
                    tunnel: w2884 -> [_ w2890]
                    tunnel: w2883 -> [_ w2889]
                    tunnel: w2882 -> [_ w2886]
                    frame False {
                    }
                    frame True {
                      n1972 = flat-sequence {
                        tunnel: w2889 -> [w2894]
                        tunnel: w2890 -> [w2895]
                        tunnel: [w2895] -> w2888
                        tunnel: [w2894] -> w2887
                        tunnel: w2886 -> [w2891]
                        tunnel: w2888 -> [w2905]
                        tunnel: w2887 -> [w2904]
                        tunnel: w2886 -> [w2913]
                        frame #0 {
                          n1973 = local read "Sample Channel\nFlow"() -> (w2893:bool)
                          n1974 = case shown="True" w2893 {
                            tunnel: "Flow ON \nduring return\nfrom dip?" -> [w2896 w2899]
                            tunnel: w2891 -> [_ w2898]
                            frame False {
                              n1975 = case shown="True" w2896 {
                                frame False {
                                }
                                frame True {
                                n1976 = property on="Sample Channel\nFlow" class="Bool (strict)"("Val(Sgnl)"=TRUE ("Value (Signaling)")) -> ()  [unwired: 2 in, 2 out]
                                }
                              }
                            }
                            frame True {
                              n1977 = case shown="False" w2899 {
                                tunnel: w2898 -> [w2900 _]
                                frame False {
                                n1978 = property on="Trap Pos. FB ON" class="Bool (strict)"("Val(Sgnl)"=w2900) -> ()  [unwired: 2 in, 2 out]
                                n1979 = property on="Sample Channel\nFlow" class="Bool (strict)"("Val(Sgnl)"=FALSE ("Value (Signaling)")) -> ()  [unwired: 2 in, 2 out]
                                }
                                frame True {
                                }
                              }
                            }
                          }
                        }
                        frame #1 {
                          # "For turning on green laser before stage reaches lower spot"
                          n1980 = case shown="True" "Green ON\nafter start\nreturn?" {
                            frame False {
                            }
                            frame True {
                              n1981 = flat-sequence {
                                frame #0 {
                                n1982 = Multiply(x="Green delay after \nstart return (s)", y=1000.0) -> (x*y=w2910:dbl)
                                n1983 = Wait (ms)(milliseconds to wait=w2910) -> ()  [unwired: 1 out]
                                }
                                frame #1 {
                                n1984 = property on="Green Laser ON" class="Bool (strict)"("Val(Sgnl)"=TRUE ("Value (Signaling)")) -> ()  [unwired: 2 in, 2 out]
                                }
                              }
                            }
                          }
                          n1985 = local read "Saved Stage Positions"() -> (w2908:dbl[][])
                          n1986 = local write "Cancel dwell"(FALSE ("Cancel dwell")) -> ()
                          n1987 = call "move to saved stage position.vi"("error in"=w2904, "Stage VISA resource name in"=w2905, "Position"="Return Stage \nPosition", "Saved Stage Positions"=w2908) -> ("error out"=w2906:errorcluster)  [unwired: 1 out]
                          n1988 = local write "Stage Control Serial Error"(w2906) -> ()
                        }
                        frame #2 {
                          n1989 = property on="Trap Pos. FB ON" class="Bool (strict)"("Val(Sgnl)"=w2913) -> ()  [unwired: 2 in, 2 out]
                          n1990 = case shown="True" "Green ON \nafter return?" {
                            frame False {
                            }
                            frame True {
                              n1991 = property on="Green Laser ON" class="Bool (strict)"("Val(Sgnl)"=TRUE ("Value (Signaling)")) -> ()  [unwired: 2 in, 2 out]
                            }
                          }
                          n1992 = case shown="True" "Move trap after return?" {
                            frame False {
                            }
                            frame True {
                              n1993 = property on="Trap Delta (MHz)" class="DigNum (strict)"("Val(Sgnl)"="Dip Trap Delta 2 (MHz)") -> ()  [unwired: 2 in, 2 out]
                            }
                          }
                          n1994 = case shown="True" "Save data after return?" {
                            frame False {
                            }
                            frame True {
                              n1995 = property on="Start Saving" class="Bool (strict)"("Val(Sgnl)"=TRUE ("Value (Signaling)")) -> ()  [unwired: 2 in, 2 out]
                            }
                          }
                          n1996 = property on="Sample Channel\nFlow" class="Bool (strict)"("Val(Sgnl)"="Flow ON\nduring daq?") -> ()  [unwired: 2 in, 2 out]
                        }
                        frame #3 {
                          n1997 = node-c288() -> (w2922:T23)  [unwired: 4 in]
                          n1998 = timed-loop {
                            timing: w2922 -> [_]
                            timing-out: [_] -> w2921
                            i -> [w2923]
                            stop <- w2925 stop-if-true
                            n1999 = node-c288() -> ()  [unwired: 1 in, 1 out]
                            n2000 = local read "Dump Beads"() -> (w2924:bool)
                            n2001 = Greater Or Equal?(x=w2923, y="Dwell Duration (s)") -> (x >= y?=w2930:bool)
                            n2002 = local read "Dip for Protein"() -> (w2927:bool)
                            n2003 = Not(x=w2927) -> (.not. x?=w2926:bool)
                            n2004 = Compound Arithmetic op=OR(w2930, "Cancel dwell", w2926) -> (w2929:bool)
                            n2005 = node-c288() -> ()  [unwired: 1 in, 1 out]
                            n2006 = Select(t=FALSE, s="Pause dwell", f=w2929) -> (s? t:f=w2932:bool)
                            n2007 = Or(x=w2932, y=w2924) -> (x .or. y?=w2925:bool)
                            "Dwell Time (s)" <- w2923
                          }
                          n2008 = node-c288(w2921) -> ()  [unwired: 1 out]
                        }
                      }
                    }
                  }
                }
                frame #4 {
                  n2009 = local read "Dip for Protein"() -> (w2942:bool)
                  n2010 = local read "Dump Beads"() -> (w2939:bool)
                  n2011 = local write "Cancel dwell"(FALSE ("Cancel dwell")) -> ()
                  n2012 = Not(x=w2942) -> (.not. x?=w2943:bool)
                  n2013 = Not(x="Cont. Repeat Dipping?") -> (.not. x?=w2945:bool)
                  n2014 = Compound Arithmetic op=OR(w2943, w2945, w2939) -> (w2941:bool)
                }
              }
            }
          }
        }
      }
      event "Profile": Value Change {
        n2015 = event-data() -> ()  [unwired: 1 in, 5 out]
        n2016 = flat-sequence {
          tunnel: w2954 -> [w2957]
          tunnel: w2953 -> [w2965]
          tunnel: [w2959] -> w2952
          tunnel: [w2958] -> w2951
          tunnel: [w2956] -> w2949
          tunnel: [w2955] -> w2946
          tunnel: w2952 -> [w2972]
          tunnel: w2951 -> [w2971]
          tunnel: [w2969] -> w2950
          tunnel: w2949 -> [w2970]
          tunnel: [w2968] -> w2948
          tunnel: [w2967] -> w2947
          tunnel: w2946 -> [w2967]
          tunnel: w2950 -> [w2976]